vi "Minhee Analysis.vi"(5 "Data type":T4 items=["AXON", "HEKA", "TEXT"], 7 "Path of File":path=path "C:/Users/KimYG/Desktop/test4.abf") -> ()   [LabVIEW 2017] (continued)
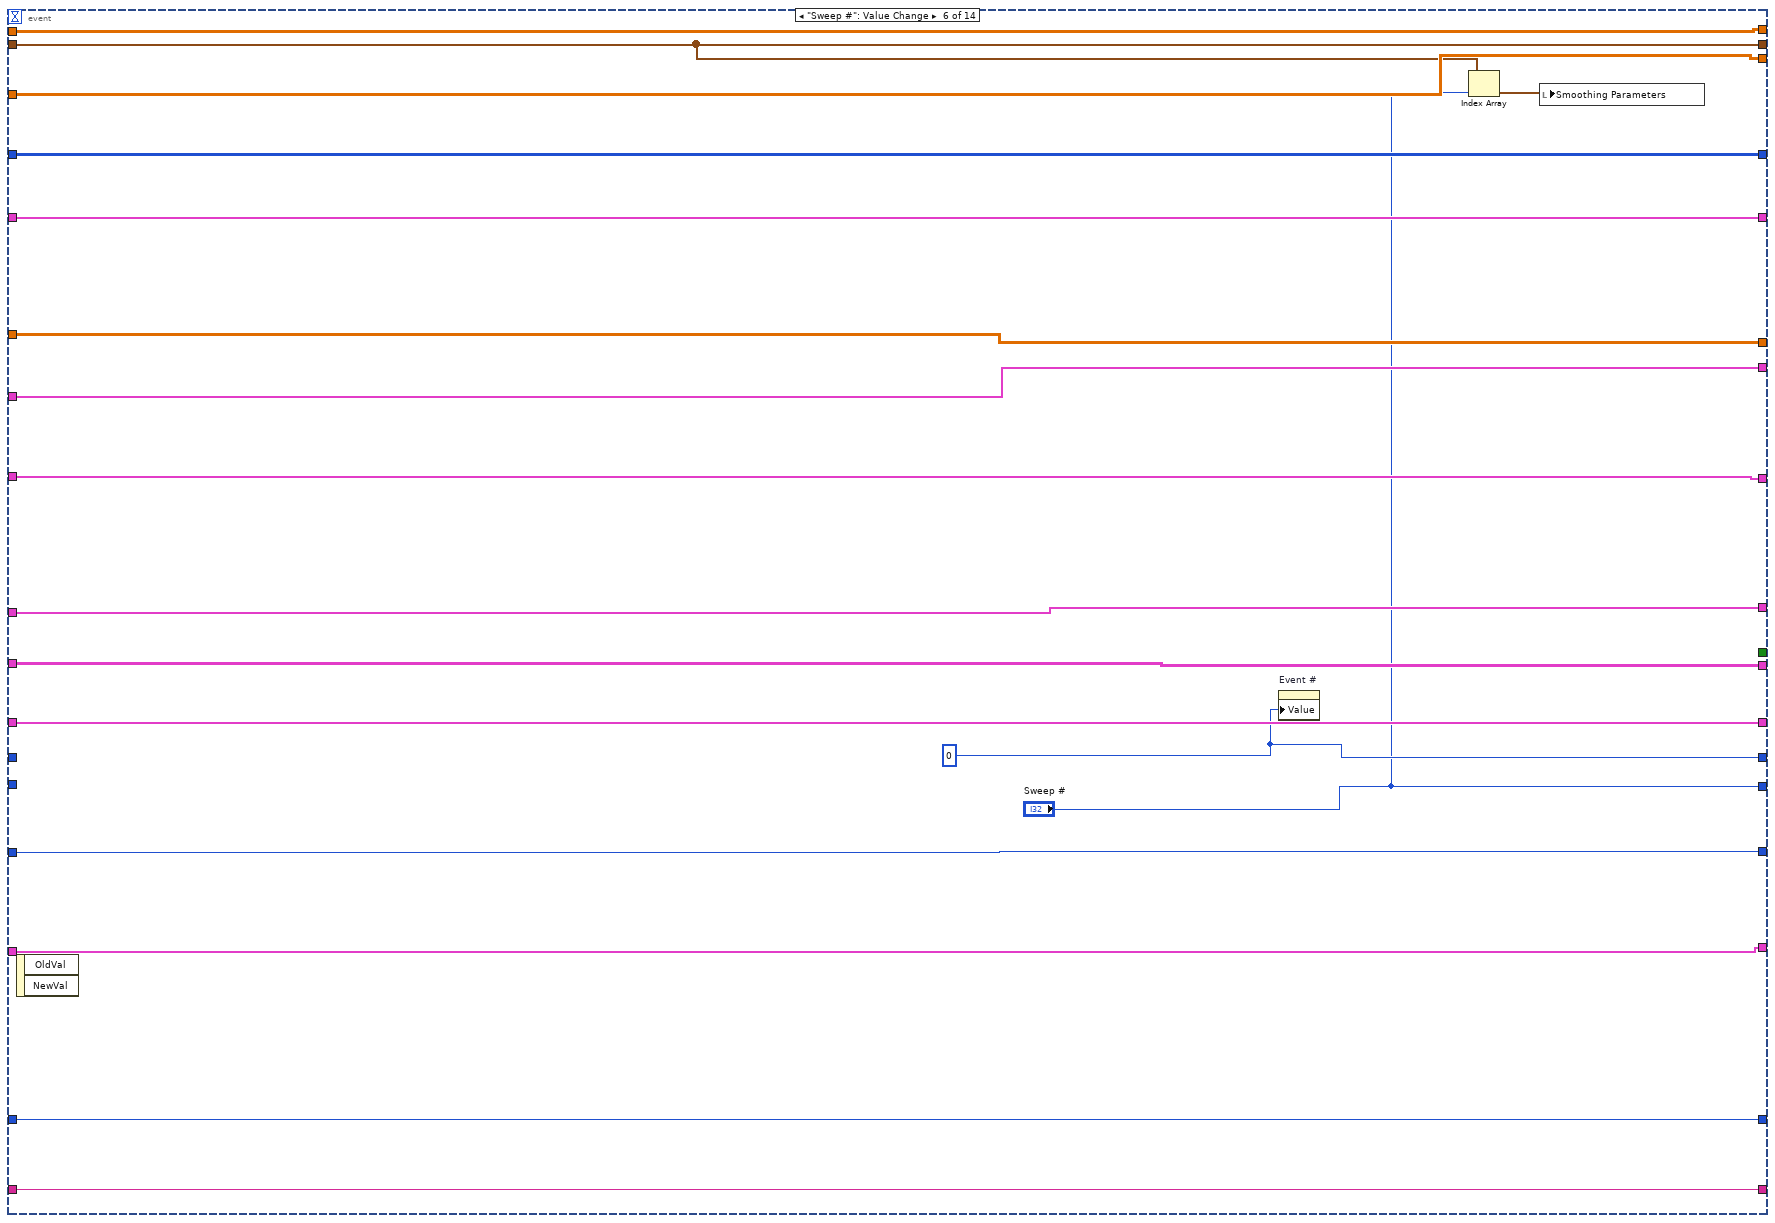
[diagram p12: hidden frame]
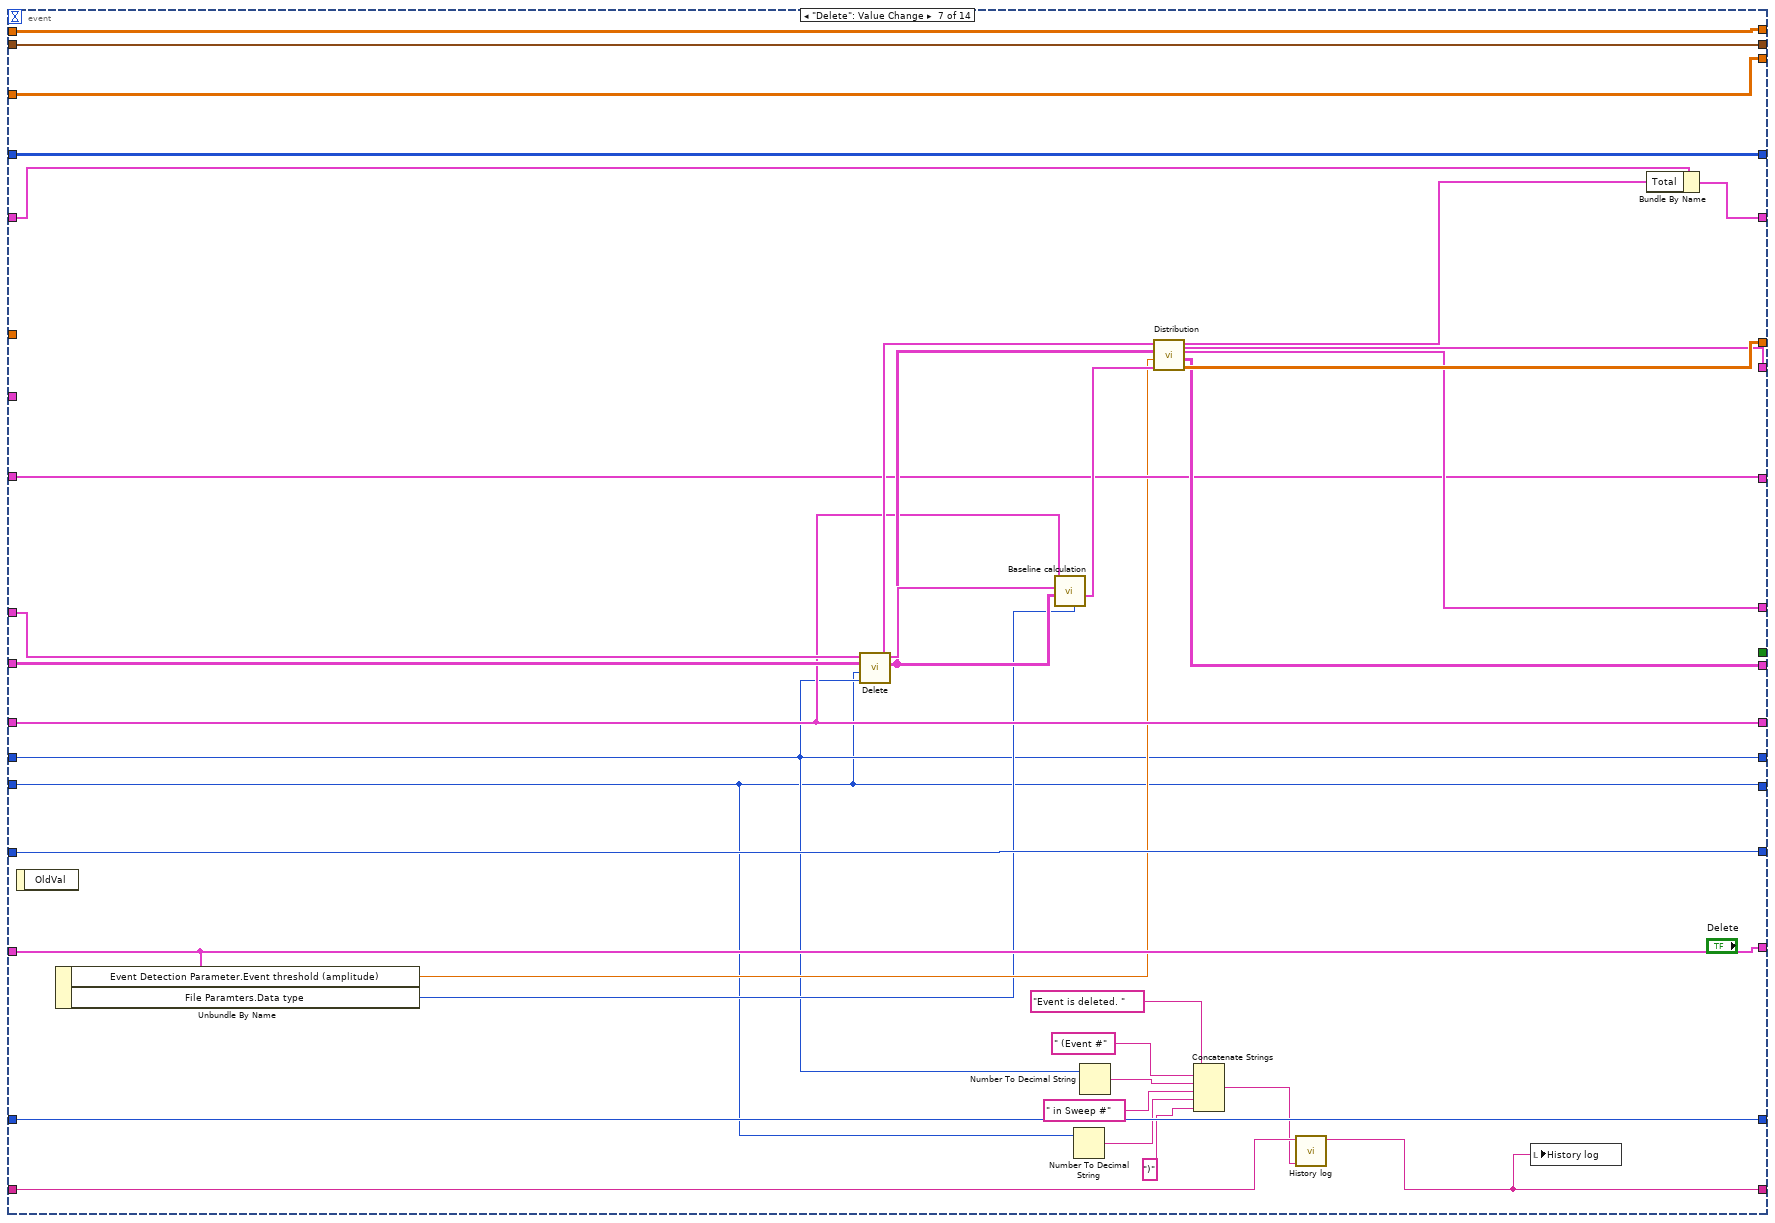
[diagram p13: hidden frame]
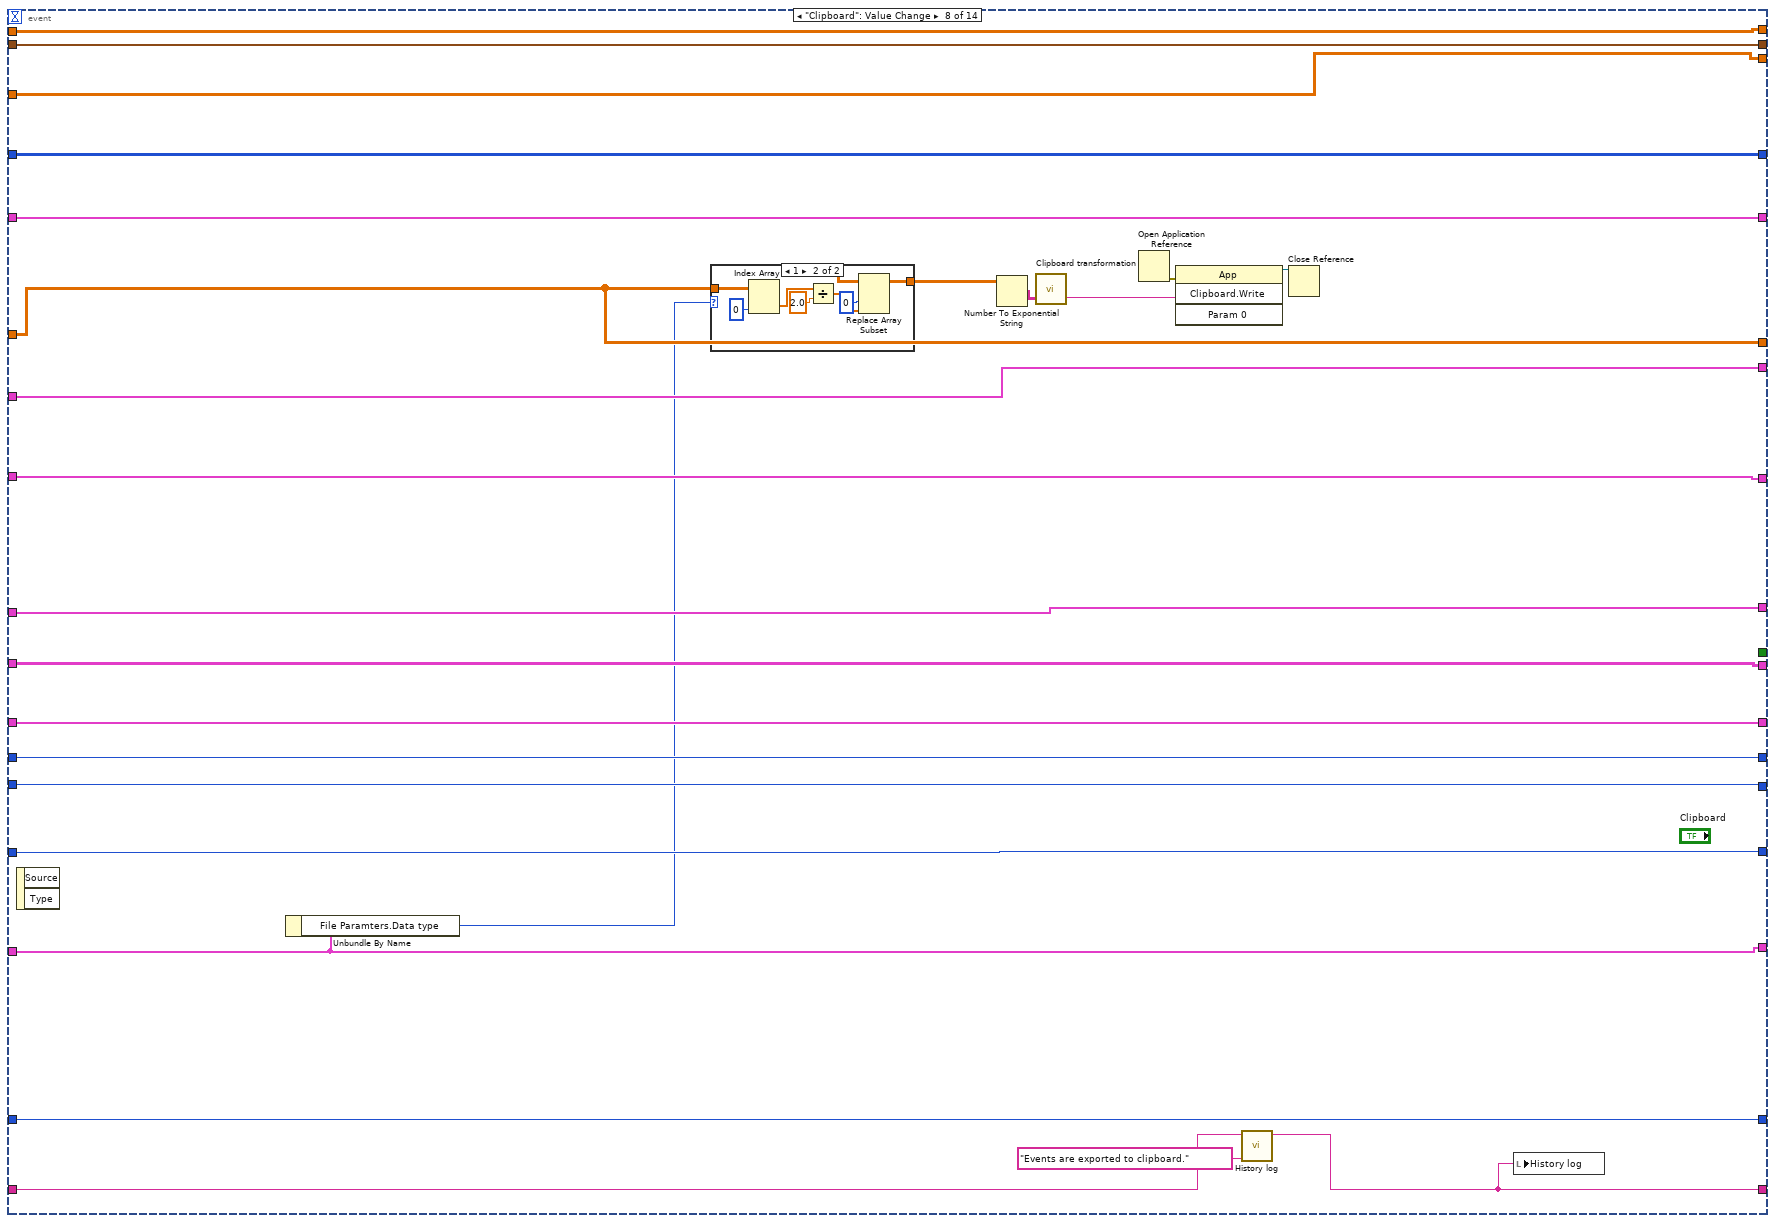
[diagram p14: hidden frame]
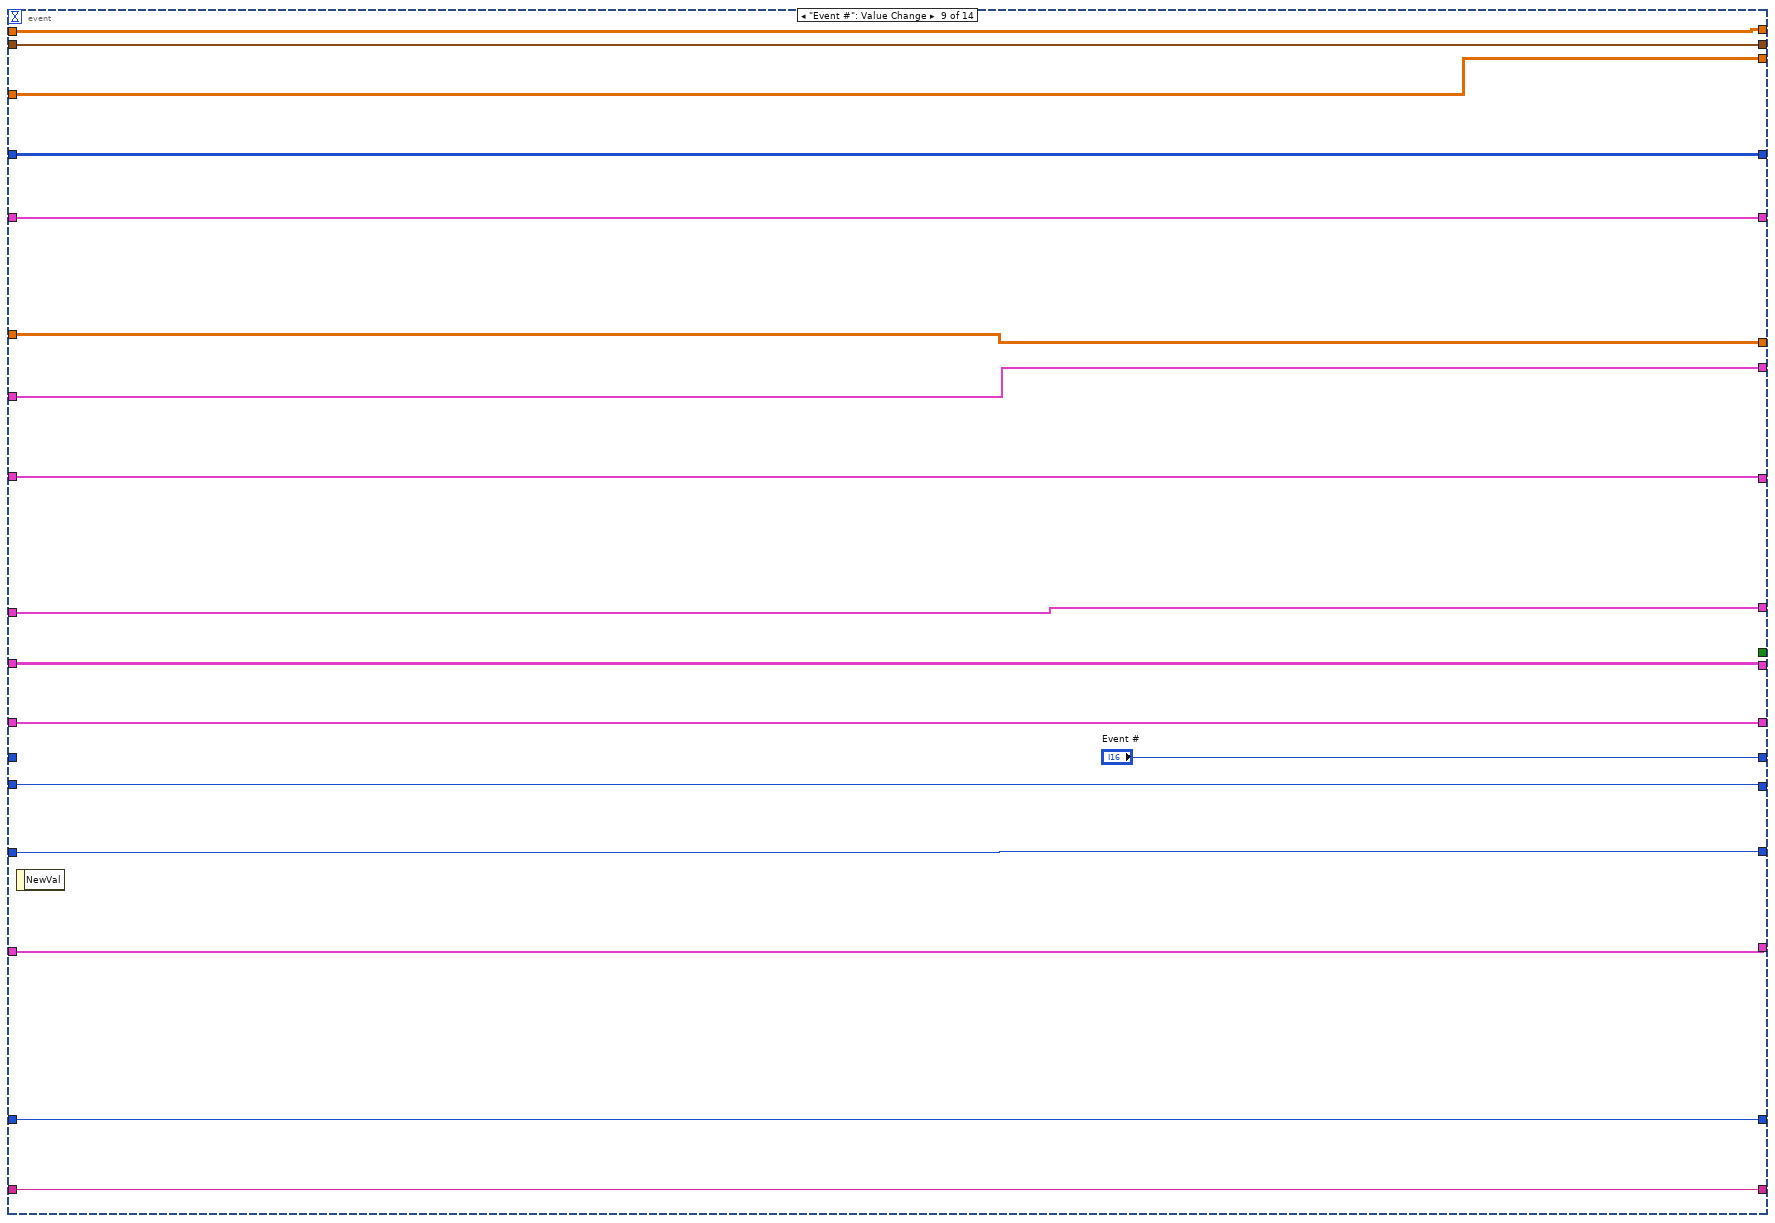
[diagram p16: hidden frame]
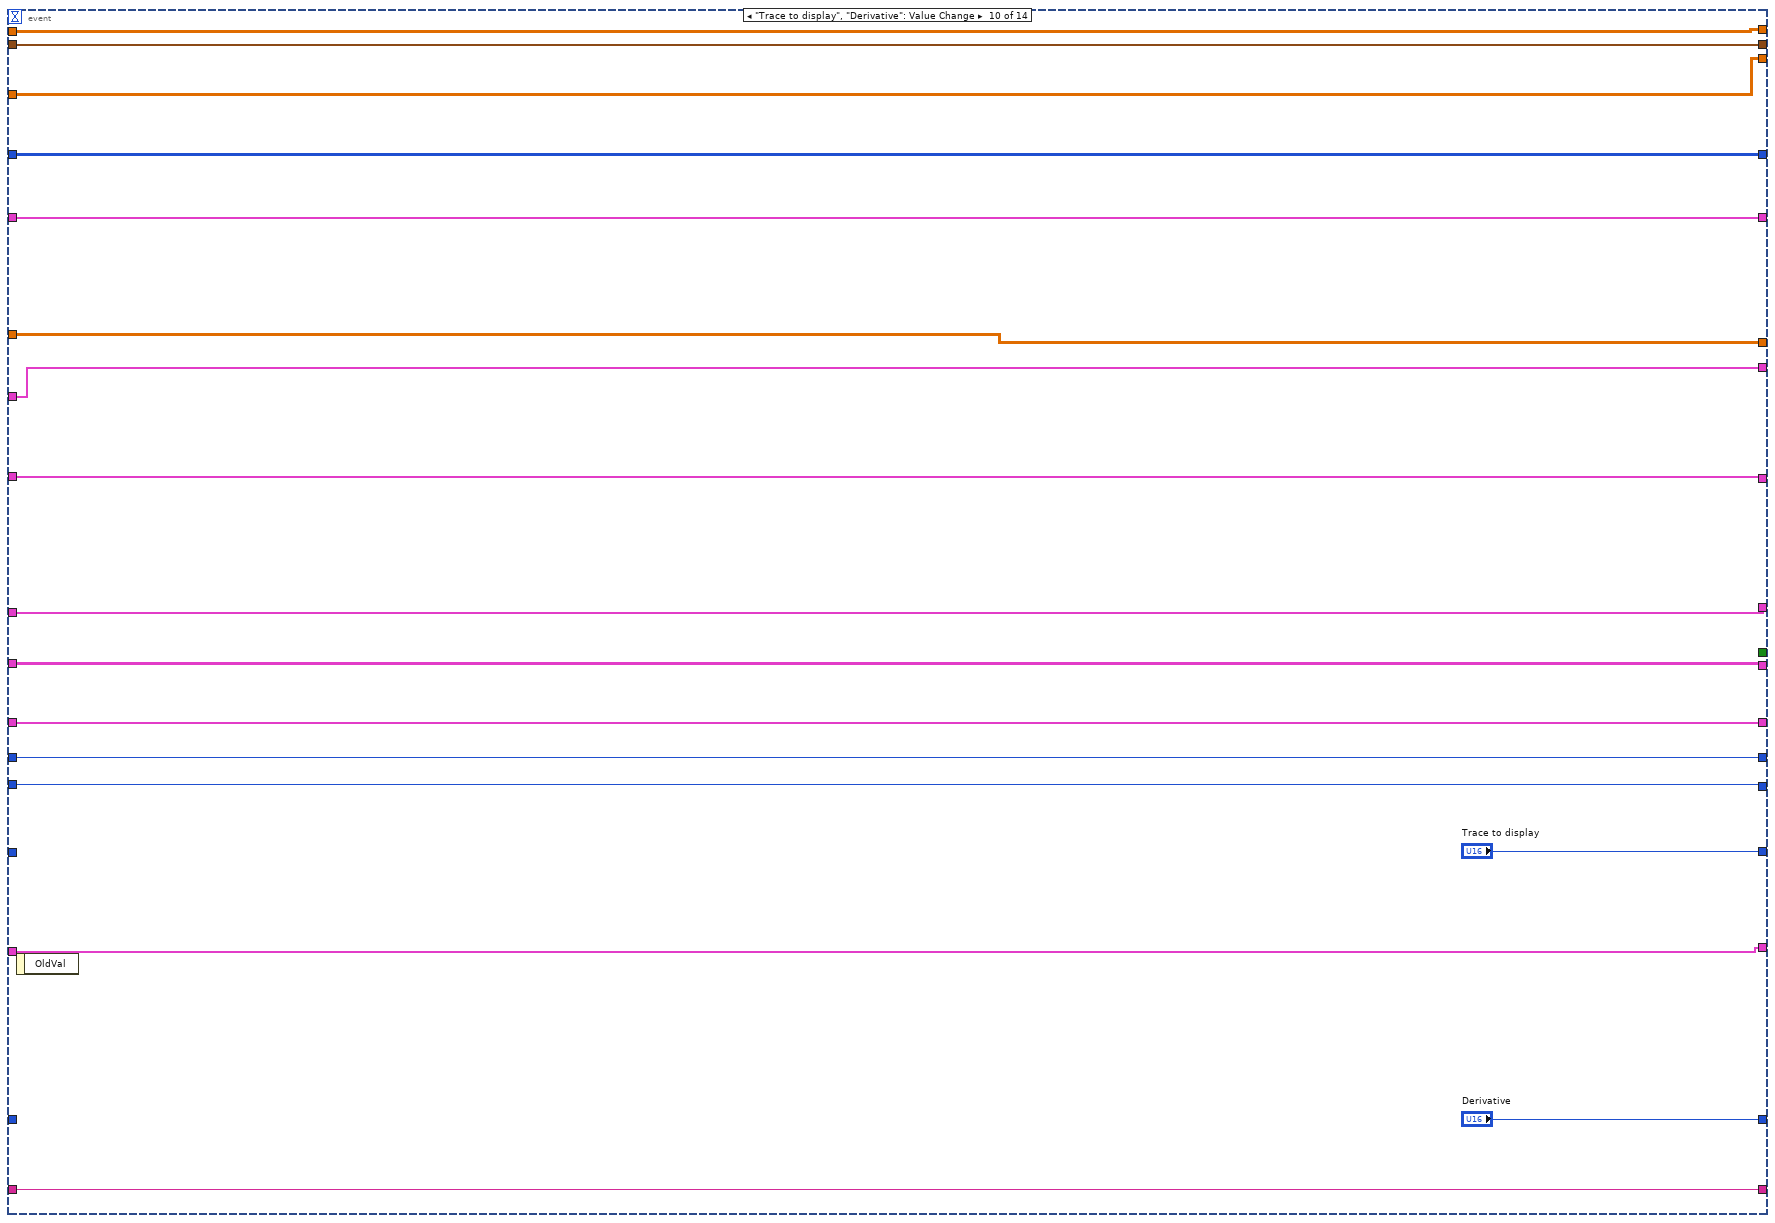
[diagram p17: hidden frame]
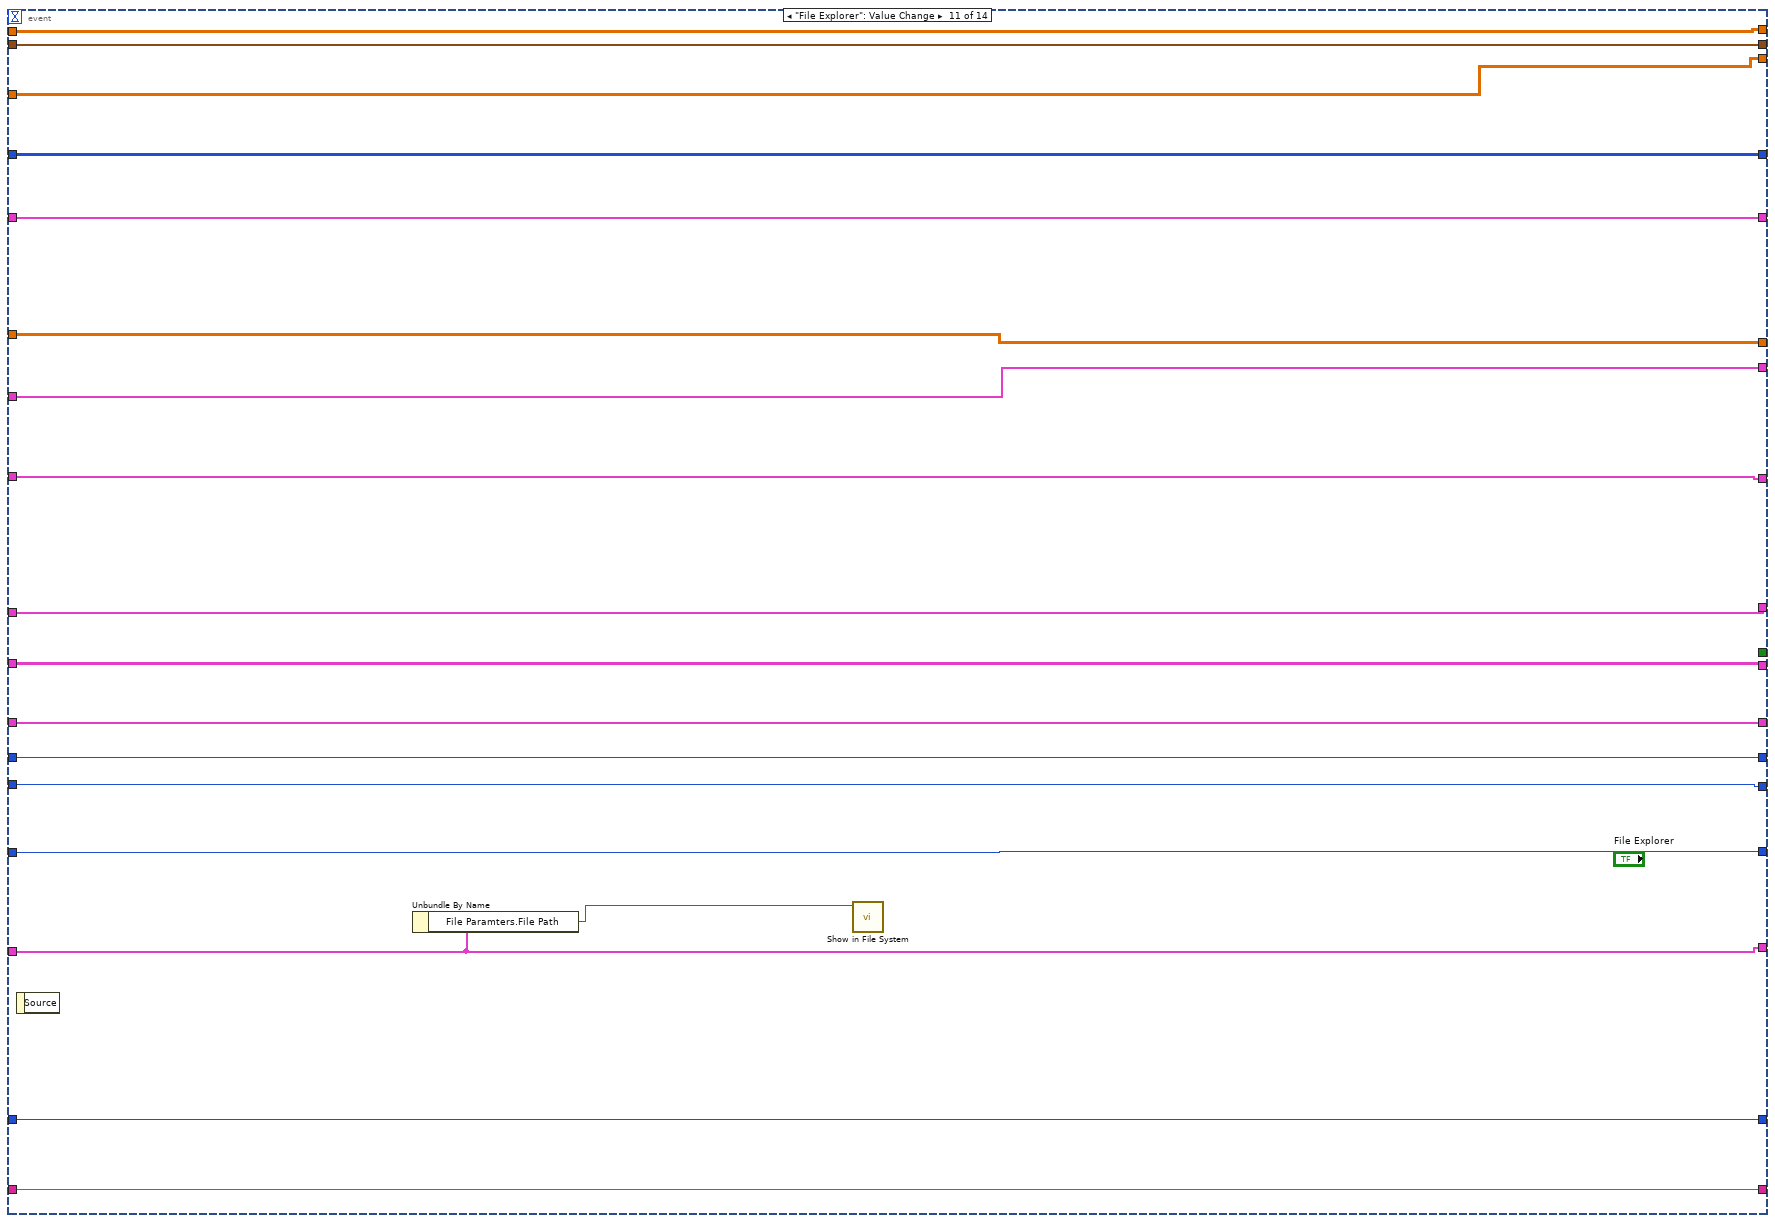
[diagram p18: hidden frame]
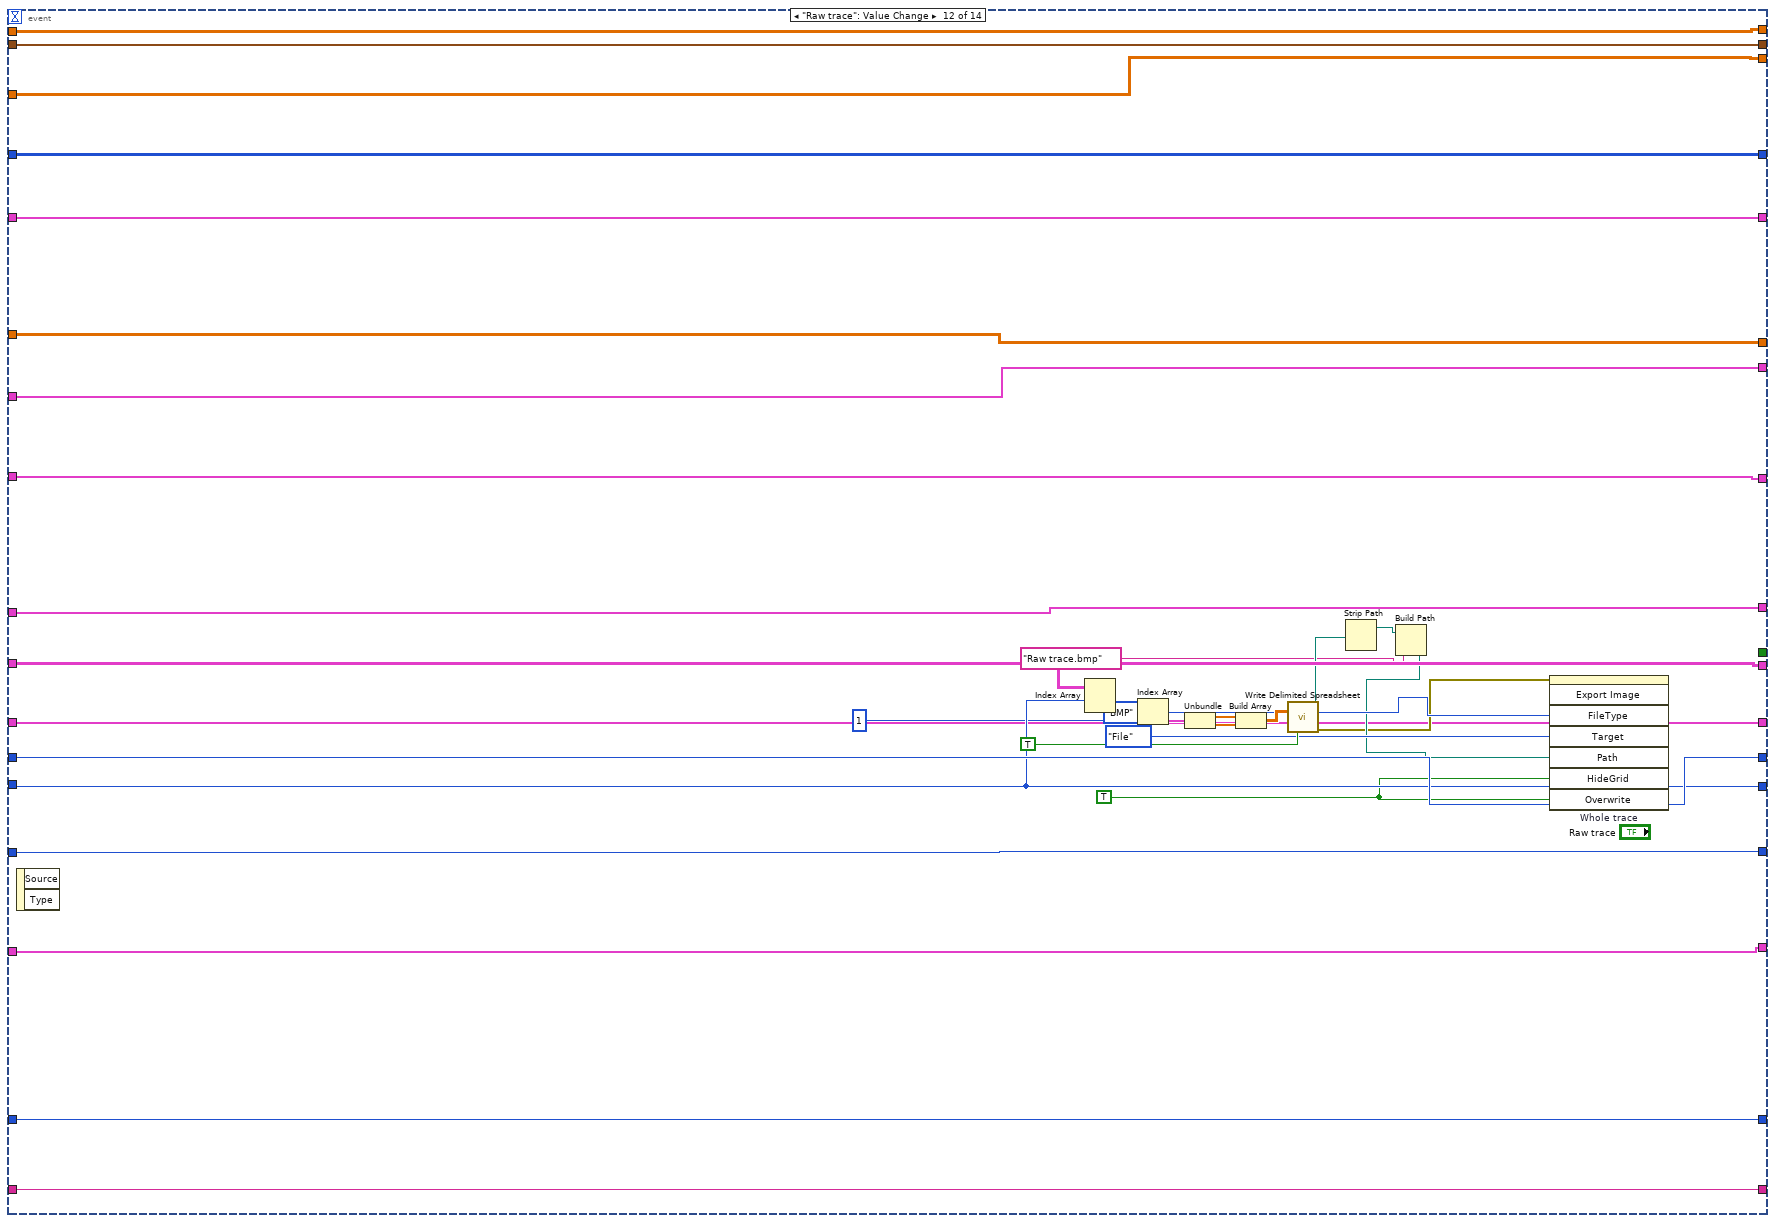
[diagram p19: hidden frame]
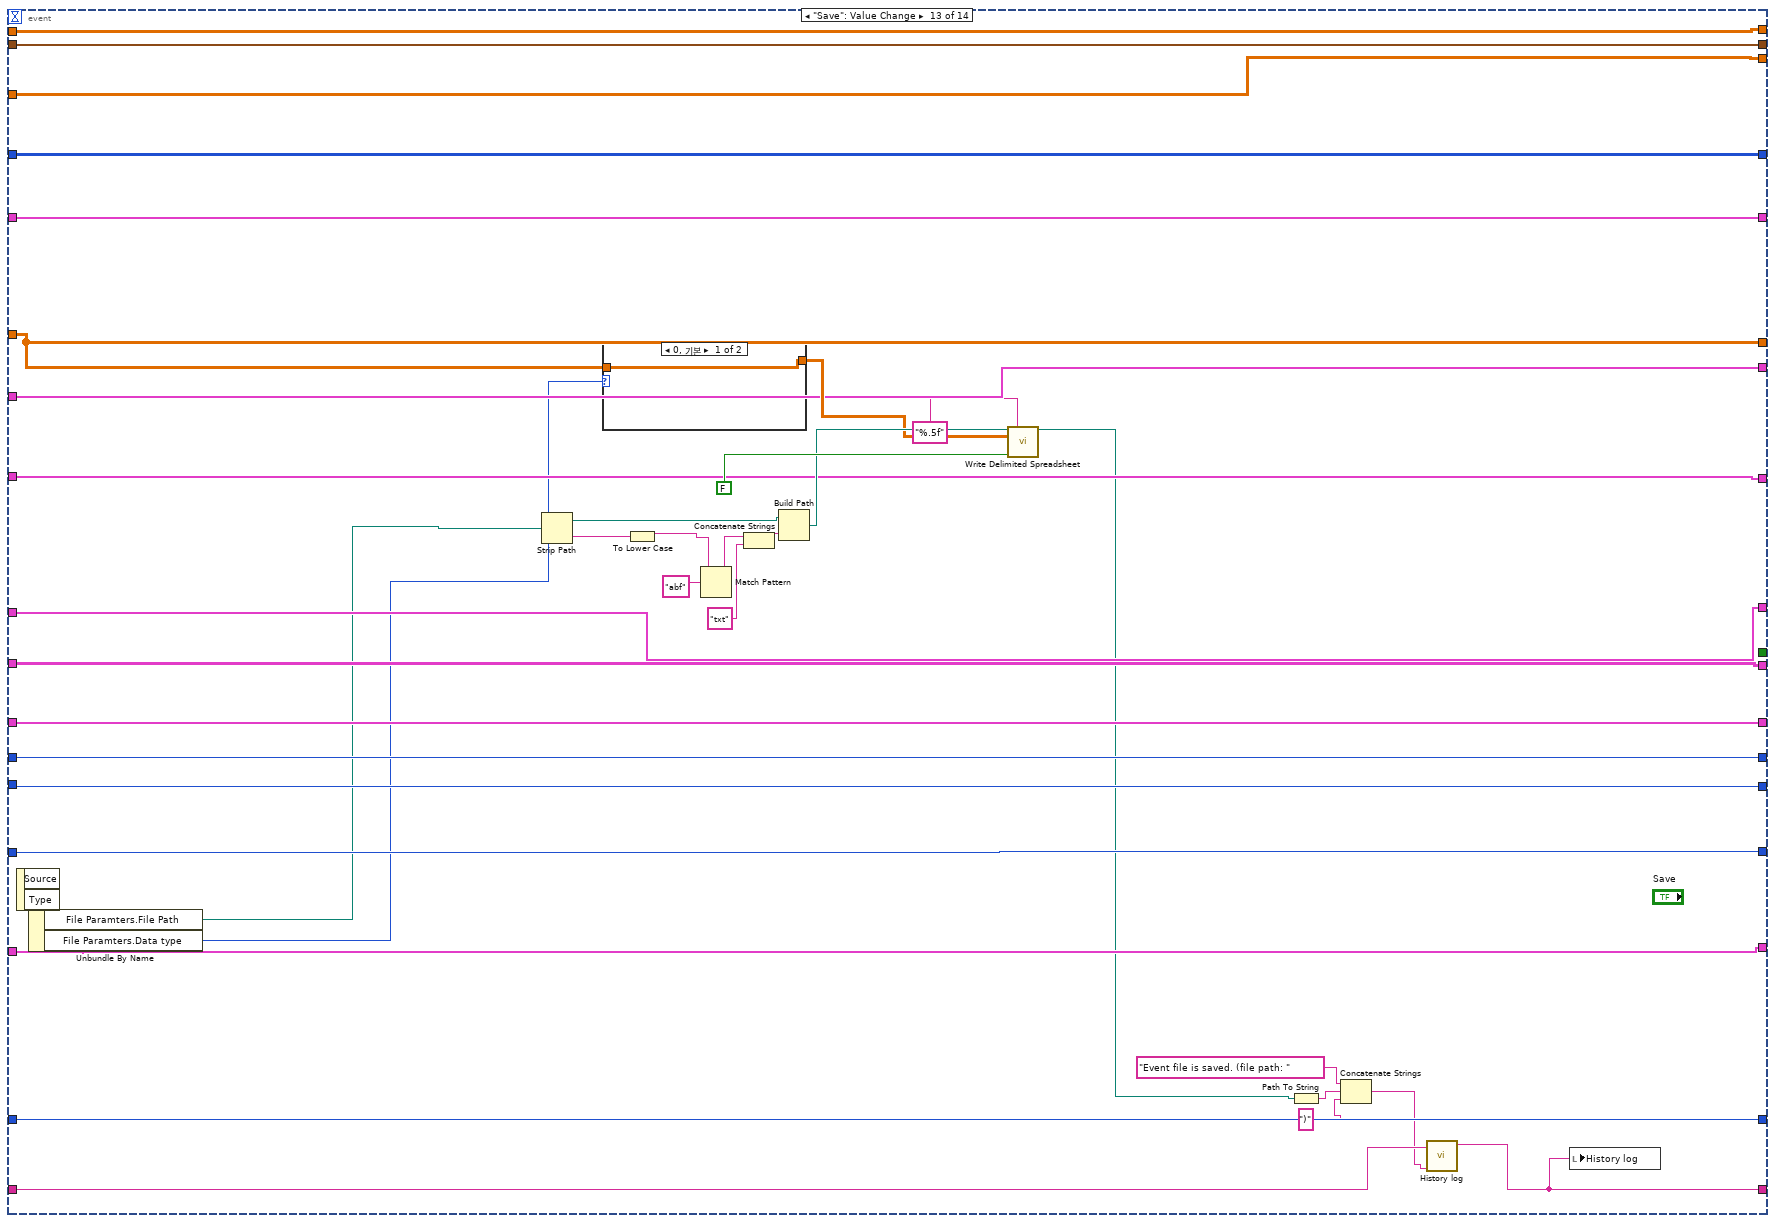
[diagram p20: hidden frame]
